vi "Dresden R2R Sputter 03.02.2018 IY24.vi"() -> ()   [LabVIEW 2009] (continued)
            n2054 = Greater?(x=w3765, y=3.0) -> (0:w3772:bool)
            n2055 = Not(x=w3772) -> (.not. x?=w3768:bool)
            n2056 = In Range and Coerce(upper limit=3.0, x=w3765, lower limit=0.0) -> (In Range?=w3764:bool)  [unwired: 1 out]
            n2057 = local write "Ch2_Ch_vbv_timer"(w3768) -> ()
            n2058 = property on="Ch_vbv_tab_ch2_gui" class="TabCtl (strict)"("Visible"=w3764) -> ()  [unwired: 2 in, 2 out]
          }
        }
        n2059 = case shown="True" w2865 {
          tunnel: w2863 -> [_ w3746]
          tunnel: [TRUE FALSE] -> w2864
          frame #0 {
          }
          frame #1 {
            n2060 = call "Elapsed Time20"("Reset"=w3746) -> ("Elapsed Time (s)"=w3745:dbl)  [unwired: 11 in, 7 out]
            n2061 = Greater?(x=w3745, y=3.0) -> (0:w3752:bool)
            n2062 = Not(x=w3752) -> (.not. x?=w3748:bool)
            n2063 = In Range and Coerce(upper limit=3.0, x=w3745, lower limit=0.0) -> (In Range?=w3744:bool)  [unwired: 1 out]
            n2064 = local write "Ch4_Ch_vbv_timer"(w3748) -> ()
            n2065 = property on="Ch_vbv_tab_ch4_gui" class="TabCtl (strict)"("Visible"=w3744) -> ()  [unwired: 2 in, 2 out]
          }
        }
        n2066 = case shown="True" w2854 {
          tunnel: w2856 -> [_ w3716]
          tunnel: [TRUE FALSE] -> w2855
          frame #0 {
          }
          frame #1 {
            n2067 = call "Elapsed Time23"("Reset"=w3716) -> ("Elapsed Time (s)"=w3715:dbl)  [unwired: 11 in, 7 out]
            n2068 = Greater?(x=w3715, y=3.0) -> (0:w3722:bool)
            n2069 = Not(x=w3722) -> (.not. x?=w3718:bool)
            n2070 = In Range and Coerce(upper limit=3.0, x=w3715, lower limit=0.0) -> (In Range?=w3714:bool)  [unwired: 1 out]
            n2071 = local write "Ch3_Tp_timer"(w3718) -> ()
            n2072 = property on="Tp_ch3_tab_gui" class="TabCtl (strict)"("Visible"=w3714) -> ()  [unwired: 2 in, 2 out]
          }
        }
        n2073 = case shown="True" w2866 {
          tunnel: w2868 -> [_ w3756]
          tunnel: [TRUE FALSE] -> w2867
          frame #0 {
          }
          frame #1 {
            n2074 = call "Elapsed Time19"("Reset"=w3756) -> ("Elapsed Time (s)"=w3755:dbl)  [unwired: 11 in, 7 out]
            n2075 = Greater?(x=w3755, y=3.0) -> (0:w3762:bool)
            n2076 = Not(x=w3762) -> (.not. x?=w3758:bool)
            n2077 = In Range and Coerce(upper limit=3.0, x=w3755, lower limit=0.0) -> (In Range?=w3754:bool)  [unwired: 1 out]
            n2078 = local write "Ch3_Ch_vbv_timer"(w3758) -> ()
            n2079 = property on="Ch_vbv_tab_ch3_gui" class="TabCtl (strict)"("Visible"=w3754) -> ()  [unwired: 2 in, 2 out]
          }
        }
        n2080 = case shown="True" w2860 {
          tunnel: w2862 -> [_ w3736]
          tunnel: [TRUE FALSE] -> w2861
          frame #0 {
          }
          frame #1 {
            n2081 = call "Elapsed Time21"("Reset"=w3736) -> ("Elapsed Time (s)"=w3735:dbl)  [unwired: 11 in, 7 out]
            n2082 = Greater?(x=w3735, y=3.0) -> (0:w3742:bool)
            n2083 = Not(x=w3742) -> (.not. x?=w3738:bool)
            n2084 = In Range and Coerce(upper limit=3.0, x=w3735, lower limit=0.0) -> (In Range?=w3734:bool)  [unwired: 1 out]
            n2085 = local write "Ch1_Tp_timer"(w3738) -> ()
            n2086 = property on="Tp_ch1_tab_gui" class="TabCtl (strict)"("Visible"=w3734) -> ()  [unwired: 2 in, 2 out]
          }
        }
        n2087 = case shown="True" w2836 {
          tunnel: w2838 -> [_ w3656]
          tunnel: [TRUE FALSE] -> w2837
          frame #0 {
          }
          frame #1 {
            n2088 = call "Elapsed Time29"("Reset"=w3656) -> ("Elapsed Time (s)"=w3655:dbl)  [unwired: 11 in, 7 out]
            n2089 = Greater?(x=w3655, y=3.0) -> (0:w3662:bool)
            n2090 = Not(x=w3662) -> (.not. x?=w3658:bool)
            n2091 = In Range and Coerce(upper limit=3.0, x=w3655, lower limit=0.0) -> (In Range?=w3654:bool)  [unwired: 1 out]
            n2092 = local write "Gv_timer_ch1_2"(w3658) -> ()
            n2093 = property on="Gv_tab_ch1_2_gui" class="TabCtl (strict)"("Visible"=w3654) -> ()  [unwired: 2 in, 2 out]
          }
        }
        n2094 = case shown="True" w2859 {
          tunnel: w2857 -> [_ w3726]
          tunnel: [TRUE FALSE] -> w2858
          frame #0 {
          }
          frame #1 {
            n2095 = call "Elapsed Time22"("Reset"=w3726) -> ("Elapsed Time (s)"=w3725:dbl)  [unwired: 11 in, 7 out]
            n2096 = Greater?(x=w3725, y=3.0) -> (0:w3732:bool)
            n2097 = Not(x=w3732) -> (.not. x?=w3728:bool)
            n2098 = In Range and Coerce(upper limit=3.0, x=w3725, lower limit=0.0) -> (In Range?=w3724:bool)  [unwired: 1 out]
            n2099 = local write "Ch2_Tp_timer"(w3728) -> ()
            n2100 = property on="Tp_ch2_tab_gui" class="TabCtl (strict)"("Visible"=w3724) -> ()  [unwired: 2 in, 2 out]
          }
        }
        n2101 = case shown="True" w2835 {
          tunnel: w2833 -> [_ w3646]
          tunnel: [TRUE FALSE] -> w2834
          frame #0 {
          }
          frame #1 {
            n2102 = call "Elapsed Time30"("Reset"=w3646) -> ("Elapsed Time (s)"=w3645:dbl)  [unwired: 11 in, 7 out]
            n2103 = Greater?(x=w3645, y=3.0) -> (0:w3652:bool)
            n2104 = Not(x=w3652) -> (.not. x?=w3648:bool)
            n2105 = In Range and Coerce(upper limit=3.0, x=w3645, lower limit=0.0) -> (In Range?=w3644:bool)  [unwired: 1 out]
            n2106 = local write "Gv_timer_ch2_3"(w3648) -> ()
            n2107 = property on="Gv_tab_ch2_3_gui" class="TabCtl (strict)"("Visible"=w3644) -> ()  [unwired: 2 in, 2 out]
          }
        }
        n2108 = case shown="True" w2829 {
          tunnel: w2827 -> [_ w3626]
          tunnel: [TRUE FALSE] -> w2828
          frame #0 {
          }
          frame #1 {
            n2109 = call "Elapsed Time32"("Reset"=w3626) -> ("Elapsed Time (s)"=w3625:dbl)  [unwired: 11 in, 7 out]
            n2110 = Greater?(x=w3625, y=3.0) -> (0:w3632:bool)
            n2111 = Not(x=w3632) -> (.not. x?=w3628:bool)
            n2112 = In Range and Coerce(upper limit=3.0, x=w3625, lower limit=0.0) -> (In Range?=w3624:bool)  [unwired: 1 out]
            n2113 = local write "Ch1_Cc_timer"(w3628) -> ()
            n2114 = property on="Cc_tab_ch1_gui" class="TabCtl (strict)"("Visible"=w3624) -> ()  [unwired: 2 in, 2 out]
          }
        }
        n2115 = case shown="True" w2830 {
          tunnel: w2832 -> [_ w3636]
          tunnel: [TRUE FALSE] -> w2831
          frame #0 {
          }
          frame #1 {
            n2116 = call "Elapsed Time31"("Reset"=w3636) -> ("Elapsed Time (s)"=w3635:dbl)  [unwired: 11 in, 7 out]
            n2117 = Greater?(x=w3635, y=3.0) -> (0:w3642:bool)
            n2118 = Not(x=w3642) -> (.not. x?=w3638:bool)
            n2119 = In Range and Coerce(upper limit=3.0, x=w3635, lower limit=0.0) -> (In Range?=w3634:bool)  [unwired: 1 out]
            n2120 = local write "Gv_timer_ch3_4"(w3638) -> ()
            n2121 = property on="Gv_tab_ch3_4gui" class="TabCtl (strict)"("Visible"=w3634) -> ()  [unwired: 2 in, 2 out]
          }
        }
        n2122 = case shown="True" w2823 {
          tunnel: w2821 -> [_ w3606]
          tunnel: [TRUE FALSE] -> w2822
          frame #0 {
          }
          frame #1 {
            n2123 = call "Elapsed Time34"("Reset"=w3606) -> ("Elapsed Time (s)"=w3605:dbl)  [unwired: 11 in, 7 out]
            n2124 = Greater?(x=w3605, y=3.0) -> (0:w3612:bool)
            n2125 = Not(x=w3612) -> (.not. x?=w3608:bool)
            n2126 = In Range and Coerce(upper limit=3.0, x=w3605, lower limit=0.0) -> (In Range?=w3604:bool)  [unwired: 1 out]
            n2127 = local write "Ch3_Cc_timer"(w3608) -> ()
            n2128 = property on="Cc_tab_ch3_gui" class="TabCtl (strict)"("Visible"=w3604) -> ()  [unwired: 2 in, 2 out]
          }
        }
        n2129 = case shown="True" w2824 {
          tunnel: w2826 -> [_ w3616]
          tunnel: [TRUE FALSE] -> w2825
          frame #0 {
          }
          frame #1 {
            n2130 = call "Elapsed Time33"("Reset"=w3616) -> ("Elapsed Time (s)"=w3615:dbl)  [unwired: 11 in, 7 out]
            n2131 = Greater?(x=w3615, y=3.0) -> (0:w3622:bool)
            n2132 = Not(x=w3622) -> (.not. x?=w3618:bool)
            n2133 = In Range and Coerce(upper limit=3.0, x=w3615, lower limit=0.0) -> (In Range?=w3614:bool)  [unwired: 1 out]
            n2134 = local write "Ch2_Cc_timer"(w3618) -> ()
            n2135 = property on="Cc_tab_ch2_gui" class="TabCtl (strict)"("Visible"=w3614) -> ()  [unwired: 2 in, 2 out]
          }
        }
        n2136 = case shown="True" w2818 {
          tunnel: w2820 -> [_ w3596]
          tunnel: [TRUE FALSE] -> w2819
          frame #0 {
          }
          frame #1 {
            n2137 = call "Elapsed Time35"("Reset"=w3596) -> ("Elapsed Time (s)"=w3595:dbl)  [unwired: 11 in, 7 out]
            n2138 = Greater?(x=w3595, y=3.0) -> (0:w3602:bool)
            n2139 = Not(x=w3602) -> (.not. x?=w3598:bool)
            n2140 = In Range and Coerce(upper limit=3.0, x=w3595, lower limit=0.0) -> (In Range?=w3594:bool)  [unwired: 1 out]
            n2141 = local write "Ch4_Cc_timer"(w3598) -> ()
            n2142 = property on="Cc_tab_ch4_gui" class="TabCtl (strict)"("Visible"=w3594) -> ()  [unwired: 2 in, 2 out]
          }
        }
        n2143 = case shown="True" w2793 {
          tunnel: w2791 -> [_ w3506]
          tunnel: [TRUE FALSE] -> w2792
          frame #0 {
          }
          frame #1 {
            n2144 = call "Elapsed Time44"("Reset"=w3506) -> ("Elapsed Time (s)"=w3505:dbl)  [unwired: 11 in, 7 out]
            n2145 = Greater?(x=w3505, y=3.0) -> (0:w3512:bool)
            n2146 = Not(x=w3512) -> (.not. x?=w3508:bool)
            n2147 = In Range and Coerce(upper limit=3.0, x=w3505, lower limit=0.0) -> (In Range?=w3504:bool)  [unwired: 1 out]
            n2148 = local write "Ch3_Trns_gv_bp2"(w3508) -> ()
            n2149 = property on="Trns_gv_bp2_ch3_gui" class="TabCtl (strict)"("Visible"=w3504) -> ()  [unwired: 2 in, 2 out]
          }
        }
        n2150 = case shown="True" w2794 {
          tunnel: w2796 -> [_ w3516]
          tunnel: [TRUE FALSE] -> w2795
          frame #0 {
          }
          frame #1 {
            n2151 = call "Elapsed Time43"("Reset"=w3516) -> ("Elapsed Time (s)"=w3515:dbl)  [unwired: 11 in, 7 out]
            n2152 = Greater?(x=w3515, y=3.0) -> (0:w3522:bool)
            n2153 = Not(x=w3522) -> (.not. x?=w3518:bool)
            n2154 = In Range and Coerce(upper limit=3.0, x=w3515, lower limit=0.0) -> (In Range?=w3514:bool)  [unwired: 1 out]
            n2155 = local write "Ch2_Trns_gv_bp2"(w3518) -> ()
            n2156 = property on="Trns_gv_bp2_ch2_gui" class="TabCtl (strict)"("Visible"=w3514) -> ()  [unwired: 2 in, 2 out]
          }
        }
        n2157 = case shown="True" w2788 {
          tunnel: w2790 -> [_ w3496]
          tunnel: [TRUE FALSE] -> w2789
          frame #0 {
          }
          frame #1 {
            n2158 = call "Elapsed Time45"("Reset"=w3496) -> ("Elapsed Time (s)"=w3495:dbl)  [unwired: 11 in, 7 out]
            n2159 = Greater?(x=w3495, y=3.0) -> (0:w3502:bool)
            n2160 = Not(x=w3502) -> (.not. x?=w3498:bool)
            n2161 = In Range and Coerce(upper limit=3.0, x=w3495, lower limit=0.0) -> (In Range?=w3494:bool)  [unwired: 1 out]
            n2162 = local write "Ch2_Trns_gv_bp"(w3498) -> ()
            n2163 = property on="Trns_gv_bp_ch2_gui" class="TabCtl (strict)"("Visible"=w3494) -> ()  [unwired: 2 in, 2 out]
          }
        }
        n2164 = case shown="True" w2817 {
          tunnel: w2815 -> [_ w3586]
          tunnel: [TRUE FALSE] -> w2816
          frame #0 {
          }
          frame #1 {
            n2165 = call "Elapsed Time36"("Reset"=w3586) -> ("Elapsed Time (s)"=w3585:dbl)  [unwired: 11 in, 7 out]
            n2166 = Greater?(x=w3585, y=3.0) -> (0:w3592:bool)
            n2167 = Not(x=w3592) -> (.not. x?=w3588:bool)
            n2168 = In Range and Coerce(upper limit=3.0, x=w3585, lower limit=0.0) -> (In Range?=w3584:bool)  [unwired: 1 out]
            n2169 = local write "Bp_bv_timer_ch1_R"(w3588) -> ()
            n2170 = property on="Bp_bv_tab_ch1 R_gui" class="TabCtl (strict)"("Visible"=w3584) -> ()  [unwired: 2 in, 2 out]
          }
        }
        n2171 = case shown="True" w2787 {
          tunnel: w2785 -> [_ w3486]
          tunnel: [TRUE FALSE] -> w2786
          frame #0 {
          }
          frame #1 {
            n2172 = call "Elapsed Time46"("Reset"=w3486) -> ("Elapsed Time (s)"=w3485:dbl)  [unwired: 11 in, 7 out]
            n2173 = Greater?(x=w3485, y=3.0) -> (0:w3492:bool)
            n2174 = Not(x=w3492) -> (.not. x?=w3488:bool)
            n2175 = In Range and Coerce(upper limit=3.0, x=w3485, lower limit=0.0) -> (In Range?=w3484:bool)  [unwired: 1 out]
            n2176 = local write "Ch3_Trns_gv_bp"(w3488) -> ()
            n2177 = property on="Trns_gv_bp_ch3_gui" class="TabCtl (strict)"("Visible"=w3484) -> ()  [unwired: 2 in, 2 out]
          }
        }
        n2178 = case shown="True" w2811 {
          tunnel: w2809 -> [_ w3566]
          tunnel: [TRUE FALSE] -> w2810
          frame #0 {
          }
          frame #1 {
            n2179 = call "Elapsed Time38"("Reset"=w3566) -> ("Elapsed Time (s)"=w3565:dbl)  [unwired: 11 in, 7 out]
            n2180 = Greater?(x=w3565, y=3.0) -> (0:w3572:bool)
            n2181 = Not(x=w3572) -> (.not. x?=w3568:bool)
            n2182 = In Range and Coerce(upper limit=3.0, x=w3565, lower limit=0.0) -> (In Range?=w3564:bool)  [unwired: 1 out]
            n2183 = local write "Bp_bv_timer_ch3_R"(w3568) -> ()
            n2184 = property on="Bp_bv_tab_ch3_R_gui" class="TabCtl (strict)"("Visible"=w3564) -> ()  [unwired: 2 in, 2 out]
          }
        }
        n2185 = case shown="True" w2799 {
          tunnel: w2797 -> [_ w3526]
          tunnel: [TRUE FALSE] -> w2798
          frame #0 {
          }
          frame #1 {
            n2186 = call "Elapsed Time42"("Reset"=w3526) -> ("Elapsed Time (s)"=w3525:dbl)  [unwired: 11 in, 7 out]
            n2187 = Greater?(x=w3525, y=3.0) -> (0:w3532:bool)
            n2188 = Not(x=w3532) -> (.not. x?=w3528:bool)
            n2189 = In Range and Coerce(upper limit=3.0, x=w3525, lower limit=0.0) -> (In Range?=w3524:bool)  [unwired: 1 out]
            n2190 = local write "Ch1_Trns_gv_bp2"(w3528) -> ()
            n2191 = property on="Trns_gv_bp2_ch1_gui" class="TabCtl (strict)"("Visible"=w3524) -> ()  [unwired: 2 in, 2 out]
          }
        }
        n2192 = case shown="True" w2800 {
          tunnel: w2802 -> [_ w3536]
          tunnel: [TRUE FALSE] -> w2801
          frame #0 {
          }
          frame #1 {
            n2193 = call "Elapsed Time41"("Reset"=w3536) -> ("Elapsed Time (s)"=w3535:dbl)  [unwired: 11 in, 7 out]
            n2194 = Greater?(x=w3535, y=3.0) -> (0:w3542:bool)
            n2195 = Not(x=w3542) -> (.not. x?=w3538:bool)
            n2196 = In Range and Coerce(upper limit=3.0, x=w3535, lower limit=0.0) -> (In Range?=w3534:bool)  [unwired: 1 out]
            n2197 = local write "Bp_bv_timer_ch4_L"(w3538) -> ()
            n2198 = property on="Bp_bv_tab_ch4_L_gui" class="TabCtl (strict)"("Visible"=w3534) -> ()  [unwired: 2 in, 2 out]
          }
        }
        n2199 = case shown="True" w2782 {
          tunnel: w2784 -> [_ w3476]
          tunnel: [TRUE FALSE] -> w2783
          frame #0 {
          }
          frame #1 {
            n2200 = call "Elapsed Time47"("Reset"=w3476) -> ("Elapsed Time (s)"=w3475:dbl)  [unwired: 11 in, 7 out]
            n2201 = Greater?(x=w3475, y=3.0) -> (0:w3482:bool)
            n2202 = Not(x=w3482) -> (.not. x?=w3478:bool)
            n2203 = In Range and Coerce(upper limit=3.0, x=w3475, lower limit=0.0) -> (In Range?=w3474:bool)  [unwired: 1 out]
            n2204 = local write "Ch4_Trns_gv_bp"(w3478) -> ()
            n2205 = property on="Trns_gv_bp_ch4_gui" class="TabCtl (strict)"("Visible"=w3474) -> ()  [unwired: 2 in, 2 out]
          }
        }
        n2206 = case shown="True" w2812 {
          tunnel: w2814 -> [_ w3576]
          tunnel: [TRUE FALSE] -> w2813
          frame #0 {
          }
          frame #1 {
            n2207 = call "Elapsed Time37"("Reset"=w3576) -> ("Elapsed Time (s)"=w3575:dbl)  [unwired: 11 in, 7 out]
            n2208 = Greater?(x=w3575, y=3.0) -> (0:w3582:bool)
            n2209 = Not(x=w3582) -> (.not. x?=w3578:bool)
            n2210 = In Range and Coerce(upper limit=3.0, x=w3575, lower limit=0.0) -> (In Range?=w3574:bool)  [unwired: 1 out]
            n2211 = local write "Bp_bv_timer_ch2_R"(w3578) -> ()
            n2212 = property on="Bp_bv_tab_ch2_R_gui" class="TabCtl (strict)"("Visible"=w3574) -> ()  [unwired: 2 in, 2 out]
          }
        }
        n2213 = case shown="True" w2806 {
          tunnel: w2808 -> [_ w3556]
          tunnel: [TRUE FALSE] -> w2807
          frame #0 {
          }
          frame #1 {
            n2214 = call "Elapsed Time39"("Reset"=w3556) -> ("Elapsed Time (s)"=w3555:dbl)  [unwired: 11 in, 7 out]
            n2215 = Greater?(x=w3555, y=3.0) -> (0:w3562:bool)
            n2216 = Not(x=w3562) -> (.not. x?=w3558:bool)
            n2217 = In Range and Coerce(upper limit=3.0, x=w3555, lower limit=0.0) -> (In Range?=w3554:bool)  [unwired: 1 out]
            n2218 = local write "Bp_bv_timer_ch2_L"(w3558) -> ()
            n2219 = property on="Bp_bv_tab_ch2_L_gui" class="TabCtl (strict)"("Visible"=w3554) -> ()  [unwired: 2 in, 2 out]
          }
        }
        n2220 = case shown="True" w2805 {
          tunnel: w2803 -> [_ w3546]
          tunnel: [TRUE FALSE] -> w2804
          frame #0 {
          }
          frame #1 {
            n2221 = call "Elapsed Time40"("Reset"=w3546) -> ("Elapsed Time (s)"=w3545:dbl)  [unwired: 11 in, 7 out]
            n2222 = Greater?(x=w3545, y=3.0) -> (0:w3552:bool)
            n2223 = Not(x=w3552) -> (.not. x?=w3548:bool)
            n2224 = In Range and Coerce(upper limit=3.0, x=w3545, lower limit=0.0) -> (In Range?=w3544:bool)  [unwired: 1 out]
            n2225 = local write "Bp_bv_timer_ch3_L"(w3548) -> ()
            n2226 = property on="Bp_bv_tab_ch3_L_gui" class="TabCtl (strict)"("Visible"=w3544) -> ()  [unwired: 2 in, 2 out]
          }
        }
        n2227 = case shown="True" w3196 {
          tunnel: w3198 -> [_ w3963]
          tunnel: w3197 -> [_ w3962]
          tunnel: [0.0 w3961] -> w2767
          frame #0 {
          }
          frame #1 {
            n2228 = Not Equal To 0?(x=w3963) -> (x != 0?=w3964:bool)
            n2229 = Less Or Equal?(x=w3963, y=30.0) -> (x <= y?=w3965:bool)
            n2230 = And(x=w3964, y=w3965) -> (x .and. y?=w3967:bool)
            n2231 = case shown="False" w3967 {
              tunnel: w3963 -> [_ w3969]
              tunnel: w3962 -> [w3968 _]
              tunnel: [w3968 w3969] -> w3961
              frame #0 {
              }
              frame #1 {
              }
            }
          }
        }
        n2232 = Add(x=w2767, y=w2769) -> (x+y=w2771:dbl)
        n2233 = Not Equal To 0?(x=w2771) -> (x != 0?=w2770:bool)
        n2234 = case shown="True" w2770 {
          tunnel: w2769 -> [_ w3458]
          tunnel: w2767 -> [_ w3459]
          tunnel: [0.0 ("y") w3457] -> w2766
          frame #0 {
          }
          frame #1 {
            n2235 = Not Equal To 0?(x=w3459) -> (x != 0?=w3462:bool)
            n2236 = Less Or Equal?(x=w3459, y=61.0) -> (x <= y?=w3463:bool)
            n2237 = And(x=w3462, y=w3463) -> (x .and. y?=w3460:bool)
            n2238 = case shown="False" w3460 {
              tunnel: w3459 -> [_ w3465]
              tunnel: w3458 -> [w3464 _]
              tunnel: [w3464 w3465] -> w3457
              frame #0 {
              }
              frame #1 {
              }
            }
          }
        }
        n2239 = case shown="48" w2766 {
          tunnel: ["" ("text") "MP" ("text") "MP" ("text") "MP" ("text") "MP" ("text") "PL-VBV" ("text") "PL-VBV" ("text") "PL-VBV" ("text") "PL-VBV" ("text") "BG-BV" ("text") "BG-BV" ("text") "BG-BV" ("text") "BG-BV" ("text") "TP-BV" ("text") "TP-BV" ("text") "TP-BV" ("text") "TP-BV" ("text") "CH-VBV" ("text") "CH-VBV" ("text") "CH-VBV" ("text") "CH-VBV" ("text") "TP" ("text") "TP" ("text") "TP" ("text") "TP" ("text") "" ("text") "" ("text") "" ("text") "" ("text") "" ("text") "" ("text") "GV-BP" ("text") "GV-BP" ("text") "GV-BP" ("text") "GV-BP" ("text") "GV-BP" ("text") "GV-BP" ("text") "PC-BV" ("text") "PC-BV" ("text") "PC-BV" ("text") "PC-BV" ("text") "GV" ("text") "GV" ("text") "GV" ("text") "CH-CC" ("text") "CH-CC" ("text") "CH-CC" ("text") "CH-CC" ("text") "PL-PG" ("text") "PL-PG" ("text") "PL-PG" ("text") "PL-PG" ("text") "PL-ATM" ("text") "PL-ATM" ("text") "PL-ATM" ("text") "PL-ATM" ("text") "CH-BG" ("text") "CH-BG" ("text") "CH-BG" ("text") "CH-BG" ("text") "CH-PG" ("text") "CH-PG" ("text") "CH-PG" ("text") "CH-PG" ("text") "CH-ATM" ("text") "CH-ATM" ("text") "CH-ATM" ("text") "CH-ATM" ("text")] -> w3352
          tunnel: [cluster{"x":i16, "y":i16} {"x"=0, "y"=0} ("origin") cluster{"x":i16, "y":i16} {"x"=1144, "y"=10} ("origin") cluster{"x":i16, "y":i16} {"x"=820, "y"=10} ("origin") cluster{"x":i16, "y":i16} {"x"=495, "y"=10} ("origin") cluster{"x":i16, "y":i16} {"x"=169, "y"=10} ("origin") cluster{"x":i16, "y":i16} {"x"=1005, "y"=160} ("origin") cluster{"x":i16, "y":i16} {"x"=678, "y"=160} ("origin") cluster{"x":i16, "y":i16} {"x"=352, "y"=160} ("origin") cluster{"x":i16, "y":i16} {"x"=35, "y"=160} ("origin") cluster{"x":i16, "y":i16} {"x"=1157, "y"=673} ("origin") cluster{"x":i16, "y":i16} {"x"=832, "y"=673} ("origin") cluster{"x":i16, "y":i16} {"x"=507, "y"=673} ("origin") cluster{"x":i16, "y":i16} {"x"=185, "y"=673} ("origin") cluster{"x":i16, "y":i16} {"x"=1070, "y"=329} ("origin") cluster{"x":i16, "y":i16} {"x"=746, "y"=329} ("origin") cluster{"x":i16, "y":i16} {"x"=420, "y"=329} ("origin") cluster{"x":i16, "y":i16} {"x"=92, "y"=329} ("origin") cluster{"x":i16, "y":i16} {"x"=1003, "y"=415} ("origin") cluster{"x":i16, "y":i16} {"x"=678, "y"=415} ("origin") cluster{"x":i16, "y":i16} {"x"=352, "y"=415} ("origin") cluster{"x":i16, "y":i16} {"x"=18, "y"=415} ("origin") cluster{"x":i16, "y":i16} {"x"=1180, "y"=373} ("origin") cluster{"x":i16, "y":i16} {"x"=859, "y"=373} ("origin") cluster{"x":i16, "y":i16} {"x"=530, "y"=373} ("origin") cluster{"x":i16, "y":i16} {"x"=202, "y"=373} ("origin") cluster{"x":i16, "y":i16} {"x"=280, "y"=243} ("origin") cluster{"x":i16, "y":i16} {"x"=606, "y"=243} ("origin") cluster{"x":i16, "y":i16} {"x"=930, "y"=243} ("origin") cluster{"x":i16, "y":i16} {"x"=358, "y"=243} ("origin") cluster{"x":i16, "y":i16} {"x"=684, "y"=243} ("origin") cluster{"x":i16, "y":i16} {"x"=1007, "y"=243} ("origin") cluster{"x":i16, "y":i16} {"x"=1031, "y"=451} ("origin") cluster{"x":i16, "y":i16} {"x"=707, "y"=451} ("origin") cluster{"x":i16, "y":i16} {"x"=385, "y"=451} ("origin") cluster{"x":i16, "y":i16} {"x"=898, "y"=451} ("origin") cluster{"x":i16, "y":i16} {"x"=571, "y"=451} ("origin") cluster{"x":i16, "y":i16} {"x"=240, "y"=451} ("origin") cluster{"x":i16, "y":i16} {"x"=1127, "y"=520} ("origin") cluster{"x":i16, "y":i16} {"x"=803, "y"=520} ("origin") cluster{"x":i16, "y":i16} {"x"=474, "y"=520} ("origin") cluster{"x":i16, "y":i16} {"x"=144, "y"=520} ("origin") cluster{"x":i16, "y":i16} {"x"=975, "y"=693} ("origin") cluster{"x":i16, "y":i16} {"x"=653, "y"=693} ("origin") cluster{"x":i16, "y":i16} {"x"=329, "y"=693} ("origin") cluster{"x":i16, "y":i16} {"x"=1094, "y"=673} ("origin") cluster{"x":i16, "y":i16} {"x"=772, "y"=673} ("origin") cluster{"x":i16, "y":i16} {"x"=445, "y"=673} ("origin") cluster{"x":i16, "y":i16} {"x"=115, "y"=673} ("origin") cluster{"x":i16, "y":i16} {"x"=248, "y"=162} ("origin") cluster{"x":i16, "y":i16} {"x"=573, "y"=162} ("origin") cluster{"x":i16, "y":i16} {"x"=903, "y"=162} ("origin") cluster{"x":i16, "y":i16} {"x"=1224, "y"=162} ("origin") cluster{"x":i16, "y":i16} {"x"=234, "y"=225} ("origin") cluster{"x":i16, "y":i16} {"x"=556, "y"=225} ("origin") cluster{"x":i16, "y":i16} {"x"=881, "y"=225} ("origin") cluster{"x":i16, "y":i16} {"x"=1207, "y"=225} ("origin") cluster{"x":i16, "y":i16} {"x"=169, "y"=801} ("origin") cluster{"x":i16, "y":i16} {"x"=493, "y"=801} ("origin") cluster{"x":i16, "y":i16} {"x"=817, "y"=801} ("origin") cluster{"x":i16, "y":i16} {"x"=1142, "y"=801} ("origin") cluster{"x":i16, "y":i16} {"x"=66, "y"=673} ("origin") cluster{"x":i16, "y":i16} {"x"=390, "y"=673} ("origin") cluster{"x":i16, "y":i16} {"x"=715, "y"=673} ("origin") cluster{"x":i16, "y":i16} {"x"=1039, "y"=673} ("origin") cluster{"x":i16, "y":i16} {"x"=270, "y"=767} ("origin") cluster{"x":i16, "y":i16} {"x"=598, "y"=767} ("origin") cluster{"x":i16, "y":i16} {"x"=922, "y"=767} ("origin") cluster{"x":i16, "y":i16} {"x"=1246, "y"=767} ("origin")] -> w3351
          tunnel: ["" ("DESCRIPTION") "Mechanical Pump" ("DESCRIPTION") "Mechanical Pump" ("DESCRIPTION") "Mechanical Pump" ("DESCRIPTION") "Mechanical Pump" ("DESCRIPTION") "Pipe Line -Vacuum Break Valve" ("DESCRIPTION") "Pipe Line -Vacuum Break Valve" ("DESCRIPTION") "Pipe Line -Vacuum Break Valve" ("DESCRIPTION") "Pipe Line -Vacuum Break Valve" ("DESCRIPTION") "Baratron Gauge-Block Valve" ("DESCRIPTION") "Baratron Gauge-Block Valve" ("DESCRIPTION") "Baratron Gauge_Block Valve" ("DESCRIPTION") "Baratron Gauge-Block Valve" ("DESCRIPTION") "Turbo Pump-Block Valve" ("DESCRIPTION") "Turbo Pump-Block Valve" ("DESCRIPTION") "Turbo Pump-Block Valve" ("DESCRIPTION") "Turbo Pump-Block Valve" ("DESCRIPTION") "Chamber Vacuum Break Valve" ("DESCRIPTION") "Chamber Vacuum Break Valve" ("DESCRIPTION") "Chamber Vacuum Break Valve" ("DESCRIPTION") "Chamber Vacuum Break Valve" ("DESCRIPTION") "Turbo Pump" ("DESCRIPTION") "Turbo Pump" ("DESCRIPTION") "Turbo Pump" ("DESCRIPTION") "Turbo Pump" ("DESCRIPTION") "" ("DESCRIPTION") "" ("DESCRIPTION") "" ("DESCRIPTION") "" ("DESCRIPTION") "" ("DESCRIPTION") "" ("DESCRIPTION") "Gate Valve- Block Valve" ("DESCRIPTION") "Gate Valve- Block Valve" ("DESCRIPTION") "Gate Valve- Block Valve" ("DESCRIPTION") "Gate Valve- Block Valve" ("DESCRIPTION") "Gate Valve- Block Valve" ("DESCRIPTION") "Gate Valve- Block Valve" ("DESCRIPTION") "Pressure Control" ("DESCRIPTION") "Pressure Control" ("DESCRIPTION") "Pressure Control" ("DESCRIPTION") "Pressure Control" ("DESCRIPTION") "Gate Valve" ("DESCRIPTION") "Gate Valve" ("DESCRIPTION") "Gate Valve" ("DESCRIPTION") "Chamber-Cold Cathode" ("DESCRIPTION") "Chamber-Cold Cathode" ("DESCRIPTION") "Chamber-Cold Cathode" ("DESCRIPTION") "Chamber-Cold Cathode" ("DESCRIPTION") "Pipe Line-Pirani Gauge" ("DESCRIPTION") "Pipe Line-Pirani Gauge" ("DESCRIPTION") "Pipe Line-Pirani Gauge" ("DESCRIPTION") "Pipe Line-Pirani Gauge" ("DESCRIPTION") "Pipe Line-Atmospheric Switch" ("DESCRIPTION") "Pipe Line-Atmospheric Switch" ("DESCRIPTION") "Pipe Line-Atmospheric Switch" ("DESCRIPTION") "Pipe Line-Atmospheric Switch" ("DESCRIPTION") "Chamber-Baratron Gauge" ("DESCRIPTION") "Chamber-Baratron Gauge" ("DESCRIPTION") "Chamber-Baratron Gauge" ("DESCRIPTION") "Chamber-Baratron Gauge" ("DESCRIPTION") "Chamber-Pirani Gauge" ("DESCRIPTION") "Chamber-Pirani Gauge" ("DESCRIPTION") "Chamber-Pirani Gauge" ("DESCRIPTION") "Chamber-Pirani Gauge" ("DESCRIPTION") "Chamber- Atmospheric Switch" ("DESCRIPTION") "Chamber- Atmospheric Switch" ("DESCRIPTION") "Chamber- Atmospheric Switch" ("DESCRIPTION") "Chamber- Atmospheric Switch" ("DESCRIPTION")] -> w3350
          frame #0 {
          }
          frame #1 {
          }
          frame #2 {
          }
          frame #3 {
          }
          frame #4 {
          }
          frame #5 {
          }
          frame #6 {
          }
          frame #7 {
          }
          frame #8 {
          }
          frame #9 {
          }
          frame #10 {
          }
          frame #11 {
          }
          frame #12 {
          }
          frame #13 {
          }
          frame #14 {
          }
          frame #15 {
          }
          frame #16 {
          }
          frame #17 {
          }
          frame #18 {
          }
          frame #19 {
          }
          frame #20 {
          }
          frame #21 {
          }
          frame #22 {
          }
          frame #23 {
          }
          frame #24 {
          }
          frame #25 {
          }
          frame #26 {
          }
          frame #27 {
          }
          frame #28 {
          }
          frame #29 {
          }
          frame #30 {
          }
          frame #31 {
          }
          frame #32 {
          }
          frame #33 {
          }
          frame #34 {
          }
          frame #35 {
          }
          frame #36 {
          }
          frame #37 {
          }
          frame #38 {
          }
          frame #39 {
          }
          frame #40 {
          }
          frame #41 {
          }
          frame #42 {
          }
          frame #43 {
          }
          frame #44 {
          }
          frame #45 {
          }
          frame #46 {
          }
          frame #47 {
          }
          frame #48 {
          }
          frame #49 {
          }
          frame #50 {
          }
          frame #51 {
          }
          frame #52 {
          }
          frame #53 {
          }
          frame #54 {
          }
          frame #55 {
          }
          frame #56 {
          }
          frame #57 {
          }
          frame #58 {
          }
          frame #59 {
          }
          frame #60 {
          }
          frame #61 {
          }
          frame #62 {
          }
          frame #63 {
          }
          frame #64 {
          }
          frame #65 {
          }
          frame #66 {
          }
          frame #67 {
          }
        }
        "DESCRIPTION" <- w3350
        n2240 = call <vilib>:"Draw Text at Point.vi"("[user-specified font]"=T35 {"Font Name:"="Bold", "Size"=18, "Strikeout?"=FALSE, "Italic?"=FALSE, "Underline?"=FALSE, "Outline?"=FALSE, "Shadow?"=FALSE, "Bold?"=TRUE}, "desired font(Application)"=T36."User-specified Font", "text"=w3352, "origin"=w3351, "picture"=w3354) -> ("new picture"=w3353:picture)  [unwired: 5 in, 1 out]
      }
      frame #2 {
        n2241 = stacked-sequence {
          frame #0 {
            # "CASETTE TRANSFER"
            n2242 = Or(x="Casette_servo_100_set", y="Casette_servo_100_auto_set") -> (x .or. y?=w4271:bool)
            n2243 = Or(x="Casette_servo_300_set", y="Casette_servo_300_auto_set") -> (x .or. y?=w4274:bool)
            n2244 = case shown="True" w4271 {
              frame #0 {
              }
              frame #1 {
                n2245 = flat-sequence {
                  frame #0 {
                    n2246 = local write "Cassette_servo_speed_value"(u16 100 ("Cassette_servo_speed_value")) -> ()
                  }
                  frame #1 {
                    n2247 = Wait (ms)(milliseconds to wait=u32 200) -> ()  [unwired: 1 out]
                  }
                  frame #2 {
                    n2248 = local write "Cassette_servo_speed_auto_set"(TRUE ("Cassette_servo_speed_auto_set")) -> ()
                  }
                }
              }
            }
            n2249 = case shown="True" w4274 {
              frame #0 {
              }
              frame #1 {
                n2250 = flat-sequence {
                  frame #0 {
                    n2251 = local write "Cassette_servo_speed_value"(u16 300 ("Cassette_servo_speed_value")) -> ()
                  }
                  frame #1 {
                    n2252 = Wait (ms)(milliseconds to wait=u32 200) -> ()  [unwired: 1 out]
                  }
                  frame #2 {
                    n2253 = local write "Cassette_servo_speed_auto_set"(TRUE ("Cassette_servo_speed_auto_set")) -> ()
                  }
                }
              }
            }
            n2254 = Or(x="Casette_servo_zero_set", y="Casette_servo_zero_auto_set") -> (x .or. y?=w4268:bool)
            n2255 = case shown="True" w4268 {
              frame #0 {
              }
              frame #1 {
                n2256 = flat-sequence {
                  frame #0 {
                    n2257 = local write "Cassette_servo_speed_value"(u16 0 ("Cassette_servo_speed_value")) -> ()
                  }
                  frame #1 {
                    n2258 = Wait (ms)(milliseconds to wait=u32 200) -> ()  [unwired: 1 out]
                  }
                  frame #2 {
                    n2259 = local write "Cassette_servo_speed_auto_set"(TRUE ("Cassette_servo_speed_auto_set")) -> ()
                  }
                  frame #3 {
                    n2260 = Wait (ms)(milliseconds to wait=u32 1000) -> ()  [unwired: 1 out]
                  }
                  frame #4 {
                    n2261 = local write "Cassette_servo_speed_auto_set"(FALSE ("Cassette_servo_speed_auto_set")) -> ()
                  }
                }
              }
            }
            n2262 = case shown="True" "Casette_start" {
              frame #0 {
              }
              frame #1 {
                n2263 = local write "Casette_servo_start/stop_do"(TRUE ("Casette_servo_start/stop_do")) -> ()
              }
            }
            n2264 = case shown="True" "Casette_stop" {
              frame #0 {
              }
              frame #1 {
                n2265 = local write "Casette_servo_start/stop_do"(FALSE ("Casette_servo_start/stop_do")) -> ()
              }
            }
          }
        }
        n2266 = stacked-sequence {
          frame #0 {
            # "SAFETY CHECK"
            n2267 = case shown="False" "Security_cancel_ch1" {
              frame #0 {
                n2268 = local read "Ch1_pressure 2"() -> (w4681:dbl)
                n2269 = local read "Ch1_Ch_atm_on"() -> (w4687:bool)
                n2270 = local read "Ch2_pressure2"() -> (w4680:dbl)
                n2271 = local read "Ar_sccm_act 5"() -> (w4660:dbl)
                n2272 = local read "Ch1_pressure 2"() -> (w4667:dbl)
                n2273 = local read "Ch2_pressure2"() -> (w4668:dbl)
                n2274 = local read "Ar_sccm_act 5"() -> (w4659:dbl)
                n2275 = local read "Ch2_Ch_atm_on"() -> (w4672:bool)
                n2276 = local read "Ch1_Ch_vbv_on"() -> (w4744:bool)
                n2277 = local read "Ch1_Ch_atm_on"() -> (w4673:bool)
                n2278 = local read "Ch1_Pl_vbv_on"() -> (w4745:bool)
                n2279 = local read "Ch1_Ch_atm_on"() -> (w4676:bool)
                n2280 = local read "ch4_sov_Ar_on_top"() -> (w4689:bool)
                n2281 = local read "Counter_read_data"() -> (w4658:i16)
                n2282 = local read "Ch1_Trns_gv_close_di"() -> (w4688:bool)
                n2283 = local read "Ch1_Ds_di"() -> (w4683:bool)
                n2284 = local read "Ch1_Tp_bv_on"() -> (w4739:bool)
                n2285 = local read "Ch1_Bg_bv_on"() -> (w4713:bool)
                n2286 = local read "Ch1_Ch_vbv_on"() -> (w4700:bool)
                n2287 = local read "Ch1_Ch_cc_on"() -> (w4715:bool)
                n2288 = local read "Ch1_Ch_atm_on"() -> (w4701:bool)
                n2289 = local read "Ch1_pressure 2"() -> (w4703:dbl)
                n2290 = local read "Ar_sccm_act 5"() -> (w4661:dbl)
                n2291 = local read "Tp1_stopped"() -> (w4726:bool)
                n2292 = local read "Ch1_Tp_bv_on"() -> (w4727:bool)
                n2293 = local read "Ch1_Ch_vbv_on"() -> (w4691:bool)
                n2294 = local read "Ch1_pressure 2"() -> (w4736:dbl)
                n2295 = local read "Ch1_Tp_bv_on"() -> (w4742:bool)
                n2296 = local read "Ch1_Mp_di"() -> (w4728:bool)
                n2297 = local read "Ch1_pressure 2"() -> (w4706:dbl)
                n2298 = local read "TP1_working"() -> (w4723:bool)
                n2299 = local read "Ch1_pressure 2"() -> (w4735:dbl)
                n2300 = local read "Ch1_Tp_bv_on"() -> (w4730:bool)
                n2301 = Less?(x=w4681, y=0.9) -> (x < y?=w4678:bool)
                n2302 = local read "Ch1_Pc_bv_on"() -> (w4708:bool)
                n2303 = local read "TP1_working"() -> (w4733:bool)
                n2304 = local read "Dcps_is_on"() -> (w4720:bool)
                n2305 = Less?(x=w4680, y=0.9) -> (x < y?=w4677:bool)
                n2306 = local read "Tp1_stopped"() -> (w4725:bool)
                n2307 = local read "Ch1_Mp_di"() -> (w4731:bool)
                n2308 = local read "TP1_working"() -> (w4709:bool)
                n2309 = Less?(x=w4667, y=0.9) -> (x < y?=w4670:bool)
                n2310 = local read "RF 1 On"() -> (w4718:bool)
                n2311 = Less?(x=w4668, y=0.9) -> (x < y?=w4671:bool)
                n2312 = case shown="False" w4687 {
                  frame #0 {
                    n2313 = local read "Ch1_Pl_atm_di"() -> (w4746:bool)
                    n2314 = case shown="False" w4746 {
                      frame #0 {
                        n2315 = local write "Ch1_Tp_bv_open_safety"(TRUE ("Tp_bv_open_ch1_safety")) -> ()
                      }
                      frame #1 {
                        n2316 = local write "Ch1_Tp_bv_open_safety"(FALSE ("Tp_bv_open_ch1_safety")) -> ()
                      }
                    }
                  }
                  frame #1 {
                    n2317 = local read "Ch1_Pl_atm_di"() -> (w4749:bool)
                    n2318 = case shown="False" w4749 {
                      frame #0 {
                        n2319 = local write "Ch1_Tp_bv_open_safety"(FALSE ("Tp_bv_open_ch1_safety")) -> ()
                      }
                      frame #1 {
                        n2320 = local write "Ch1_Tp_bv_open_safety"(TRUE ("Tp_bv_open_ch1_safety")) -> ()
                      }
                    }
                  }
                }
                n2321 = Compound Arithmetic op=OR(w4745, w4744) -> (w4743:bool)
                n2322 = Not(x=w4715) -> (.not. x?=w4714:bool)
                n2323 = Not(x=w4713) -> (.not. x?=w4712:bool)
                n2324 = And(x=w4673, y=w4672) -> (x .and. y?=w4665:bool)
                n2325 = Not(x=w4739) -> (.not. x?=w4738:bool)
                n2326 = Not(x=w4689) -> (.not. x?=w4690:bool)
                n2327 = Less?(x=w4703, y=0.1) -> (x < y?=w4699:bool)
                n2328 = Not(x=w4743) -> (.not. x?=w4685:bool)
                n2329 = Less?(x=w4659, y=0.08) -> (x < y?=w4704:bool)
                n2330 = Not And(1:w4700, 2:w4701) -> (0:w4698:bool)
                n2331 = And(x=w4678, y=w4677) -> (x .and. y?=w4675:bool)
                n2332 = Less?(x=w4660, y=0.08) -> (x < y?=w4695:bool)
                n2333 = Not Or(1:w4727, 2:w4728) -> (0:w4740:bool)
                n2334 = And(x=w4670, y=w4671) -> (x .and. y?=w4664:bool)
                n2335 = Less?(x=w4736, y=0.01) -> (x < y?=w4724:bool)
                n2336 = Less?(x=w4658, y=i16 0) -> (x < y?=w4656:bool)
                n2337 = Less?(x=w4661, y=0.08) -> (x < y?=w4722:bool)
                n2338 = Less Or Equal?(x=w4735, y=9e-05) -> (x <= y?=w4710:bool)
                n2339 = Less?(x=w4706, y=1.0) -> (x < y?=w4694:bool)
                n2340 = Not(x=w4691) -> (.not. x?=w4692:bool)
                n2341 = Not(x=w4742) -> (.not. x?=w4741:bool)
                n2342 = Not(x=w4733) -> (.not. x?=w4721:bool)
                n2343 = Not(x=w4720) -> (.not. x?=w4719:bool)
                n2344 = Not(x=w4718) -> (.not. x?=w4717:bool)
                n2345 = And(x=w4699, y=w4698) -> (x .and. y?=w4697:bool)
                n2346 = Or(x=w4676, y=w4675) -> (x .or. y?=w4674:bool)
                n2347 = And(x=w4685, y=w4683) -> (x .and. y?=w4684:bool)
                n2348 = Or(x=w4665, y=w4664) -> (x .or. y?=w4663:bool)
                n2349 = Compound Arithmetic op=AND(w4694, w4692) -> (w4693:bool)
                n2350 = Compound Arithmetic op=AND(w4738, w4726, w4714, w4712, w4690, w4688) -> (w4737:bool)
                n2351 = local write "Ch1_Mp_stop_safety"(w4741) -> ()
                n2352 = Compound Arithmetic op=AND(w4730, w4731) -> (w4729:bool)
                n2353 = Compound Arithmetic op=AND(w4724, w4723, w4722) -> (w4711:bool)
                n2354 = local write "Ch1_Tp_bv_close_safety"(w4725) -> ()
                n2355 = local write "Ch1_Pl_vbv_open_safety"(w4740) -> ()
                n2356 = Compound Arithmetic op=AND(w4710, w4709, w4708) -> (→"started_up_ch1":bool)
                n2357 = Compound Arithmetic op=AND(w4721, w4719, w4717) -> (w4716:bool)
                n2358 = local write "Ch1_sov_Ar_open_safety"(w4697) -> ()
                n2359 = local write "Ch1_Trns_gv_bp2_open_safety"(w4674) -> ()
                n2360 = local write "Ch1_sov_Ar_close_safety"(w4695) -> ()
                n2361 = local write "Ch1_Bg_bv_close_safety"(w4704) -> ()
                n2362 = local write "Ch1_Bg_bv_open_safety"(w4693) -> ()
                n2363 = local write "Gv_close_ch1_2_safety"(w4656) -> ()
                n2364 = local write "Ch1_Mp_start_safety"(w4684) -> ()
                n2365 = local write "Ch1_Ch_vbv_open_safety"(w4737) -> ()
                n2366 = local write "Ch1_Cc_open_safety"(w4711) -> ()
                n2367 = local write "Gv_open_ch1_2_safety"(w4663) -> ()
                n2368 = local write "Ch1_Tp_start_safety"(w4729) -> ()
                n2369 = local write "WFC_ch1_close_safety"(w4716) -> ()
              }
              frame #1 {
                w4752 = TRUE
                "Ch1_Bg_bv_open_safety" <- w4752
                "Ch1_Bg_bv_close_safety" <- w4752
                "Ch1_Tp_bv_open_safety" <- w4752
                "Ch1_Tp_bv_close_safety" <- w4752
                "Ch1_Ch_vbv_open_safety" <- w4752
                "Ch1_Ch_vbv_close_safety" <- w4752
                "Ch1_Bp_bv_open_R_safety" <- w4752
                "Ch1_Bp_bv_close_R_safety" <- w4752
                "Ch1_Trns_gv_bp2_open_safety" <- w4752
                "Ch1_Trns_gv_bp2_close_safety" <- w4752
                "Ch1_Mp_start_safety" <- w4752
                "Ch1_Mp_stop_safety" <- w4752
                "Ch1_Pl_vbv_open_safety" <- w4752
                "Ch1_sov_Ar_open_safety" <- w4752
                "Ch1_sov_Ar_close_safety" <- w4752
                "Ch1_Cc_open_safety" <- w4752
                "Ch1_Cc_close_safety" <- w4752
                "Ch1_Tp_start_safety" <- w4752
                "Ch1_Tp_stop_safety" <- w4752
                "WFC_ch1_close_safety" <- w4752
                "Gv_open_ch1_2_safety" <- w4752
                "Gv_close_ch1_2_safety" <- w4752
              }
            }
            n2370 = case shown="False" "Security_cancel_ch2" {
              frame #0 {
                n2371 = local read "Ch2_Ch_atm_on"() -> (w4595:bool)
                n2372 = local read "Ch2_pressure2"() -> (w4578:dbl)
                n2373 = local read "Ch3_pressure2"() -> (w4579:dbl)
                n2374 = local read "Ch2_pressure2"() -> (w4575:dbl)
                n2375 = local read "Ch1_pressure 2"() -> (w4574:dbl)
                n2376 = local read "Ch3_pressure2"() -> (w4563:dbl)
                n2377 = local read "Ch2_pressure2"() -> (w4562:dbl)
                n2378 = local read "Ch2_Ch_atm_on"() -> (w4583:bool)
                n2379 = local read "Ch2_Ch_atm_on"() -> (w4558:bool)
                n2380 = local read "Ar_sccm_act 6"() -> (w4554:dbl)
                n2381 = local read "Ch3_Ch_atm_on"() -> (w4557:bool)
                n2382 = local read "Ch2_Ch_atm_on"() -> (w4570:bool)
                n2383 = local read "Ar_sccm_act 6"() -> (w4555:dbl)
                n2384 = local read "Ch2_pressure"() -> (w4626:dbl)
                n2385 = local read "Ar_sccm_act 6"() -> (w4556:dbl)
                n2386 = local read "Ch2_Ch_vbv_on"() -> (w4601:bool)
                n2387 = local read "Ch2_pressure"() -> (w4625:dbl)
                n2388 = local read "Ch2_Ch_atm_on"() -> (w4600:bool)
                n2389 = local read "Ch2_Tp_bv_on"() -> (w4634:bool)
                n2390 = local read "Ch2_Tp_bv_on"() -> (w4638:bool)
                n2391 = local read "Ch2_Ch_vbv_on"() -> (w4591:bool)
                n2392 = local read "Ch2_Tp_bv_on"() -> (w4628:bool)
                n2393 = local read "Ch2_Ch_vbv_on"() -> (w4640:bool)
                n2394 = local read "Ch2_pressure"() -> (w4598:dbl)
                n2395 = local read "Ch2_Pl_vbv_on"() -> (w4641:bool)
                n2396 = local read "TP2_working"() -> (w4621:bool)
                n2397 = local read "Ch2_Tp_bv_on"() -> (w4648:bool)
                n2398 = local read "Ch2_Bg_bv_on"() -> (w4646:bool)
                n2399 = local read "Tp2_stopped"() -> (w4636:bool)
                n2400 = local read "TP2_working"() -> (w4623:bool)
                n2401 = local read "Ch2_Ch_cc_on"() -> (w4647:bool)
                n2402 = local read "Dcps_is_on"() -> (w4611:bool)
                n2403 = local read "TP2_working"() -> (w4616:bool)
                n2404 = local read "Ch2_Pc_bv_on"() -> (w4615:bool)
                n2405 = local read "Ch2_Mp_di"() -> (w4629:bool)
                n2406 = local read "Tp2_stopped"() -> (w4607:bool)